vi "Project-SmartHome.vi"() -> ()   [LabVIEW 2013] (continued)
      }
      event Value Change {
        # "Air conditional - Bed room (set temperature)"
        n177 = event-data() -> ()  [unwired: 1 in, 6 out]
        n178 = Decimal String To Number(string="String") -> (number=w653:i32)  [unwired: 2 in, 1 out]
        n179 = Type Cast(x=6.0) -> (*(type *) &x=w659:string)  [unwired: 1 in]
        n180 = TCP Write(connection ID=w658, data in=w659, error in (no error)=w657) -> (connection ID out=w661:refnum<k5>, error out=w662:errorcluster)  [unwired: 1 in, 1 out]
        n181 = Bundle("?", w653, 1.0) -> (w663:cluster{bool, i32, dbl})  [unwired: 1 in]
        n182 = Type Cast(x=w663) -> (*(type *) &x=w665:string)  [unwired: 1 in]
        n183 = TCP Write(connection ID=w661, data in=w665, error in (no error)=w662) -> (connection ID out=w656:refnum<k5>, error out=w655:errorcluster)  [unwired: 1 in, 1 out]
      }
      event Value Change {
        n184 = event-data() -> ()  [unwired: 1 in, 6 out]
        n185 = Type Cast(x=0.0) -> (*(type *) &x=w671:string)  [unwired: 1 in]
        n186 = TCP Write(connection ID=w668, data in=w671, error in (no error)=w669) -> (connection ID out=w667:refnum<k5>, error out=w666:errorcluster)  [unwired: 1 in, 1 out]
        n187 = Bundle("?", 15.0) -> (w675:cluster{bool, dbl})  [unwired: 1 in]
        n188 = Type Cast(x=w675) -> (*(type *) &x=w677:string)  [unwired: 1 in]
        n189 = TCP Write(connection ID=w667, data in=w677, error in (no error)=w666) -> (connection ID out=w674:refnum<k5>, error out=w673:errorcluster)  [unwired: 1 in, 1 out]
      }
      event "OK Button 18": Value Change {
        n190 = event-data() -> ()  [unwired: 1 in, 6 out]
        n191 = Type Cast(x=0.0) -> (*(type *) &x=w683:string)  [unwired: 1 in]
        n192 = TCP Write(connection ID=w680, data in=w683, error in (no error)=w681) -> (connection ID out=w679:refnum<k5>, error out=w678:errorcluster)  [unwired: 1 in, 1 out]
        n193 = Bundle("OK Button 18"="OK Button 18", 16.0) -> (w687:cluster{"OK Button 18":bool, dbl})  [unwired: 1 in]
        n194 = Type Cast(x=w687) -> (*(type *) &x=w689:string)  [unwired: 1 in]
        n195 = TCP Write(connection ID=w679, data in=w689, error in (no error)=w678) -> (connection ID out=w686:refnum<k5>, error out=w685:errorcluster)  [unwired: 1 in, 1 out]
      }
      event Value Change {
        # "Air conditional - Bedroom 2"
        n196 = event-data() -> ()  [unwired: 1 in, 6 out]
        n197 = property on="Tab Control" class="TabCtl (strict)"("Visible"=FALSE) -> ()  [unwired: 2 in, 2 out]
        n198 = property on="Tab Control 2" class="TabCtl (strict)"("Visible"=FALSE) -> ()  [unwired: 2 in, 2 out]
        n199 = property on="Tab Control 3" class="TabCtl (strict)"("Visible"=FALSE) -> ()  [unwired: 2 in, 2 out]
        n200 = property on="Tab Control 4" class="TabCtl (strict)"("Visible"=FALSE) -> ()  [unwired: 2 in, 2 out]
        n201 = property on="Tab Control 5" class="TabCtl (strict)"("Visible"=FALSE) -> ()  [unwired: 2 in, 2 out]
        n202 = property on="Tab Control 11" class="TabCtl (strict)"("Visible"=FALSE) -> ()  [unwired: 2 in, 2 out]
        n203 = property on="Tab Control 6" class="TabCtl (strict)"("Visible"=FALSE) -> ()  [unwired: 2 in, 2 out]
        n204 = property on="Tab Control 10" class="TabCtl (strict)"("Visible"=FALSE) -> ()  [unwired: 2 in, 2 out]
        n205 = property on="Tab Control 13" class="TabCtl (strict)"("Visible"=FALSE) -> ()  [unwired: 2 in, 2 out]
        n206 = property on="Tab Control 7" class="TabCtl (strict)"("Visible"=FALSE) -> ()  [unwired: 2 in, 2 out]
        n207 = property on="Tab Control 12" class="TabCtl (strict)"("Visible"=FALSE) -> ()  [unwired: 2 in, 2 out]
        n208 = property on="Tab Control 8" class="TabCtl (strict)"("Visible"=FALSE) -> ()  [unwired: 2 in, 2 out]
        n209 = property on="Tab Control 9" class="TabCtl (strict)"("Visible"=FALSE) -> ()  [unwired: 2 in, 2 out]
        n210 = property on="Tab Control 24" class="TabCtl (strict)"("Visible"=FALSE) -> ()  [unwired: 2 in, 2 out]
        n211 = property on="Tab Control 15" class="TabCtl (strict)"("Visible"=FALSE) -> ()  [unwired: 2 in, 2 out]
        n212 = property on="Tab Control 21" class="TabCtl (strict)"("Visible"=TRUE) -> ()  [unwired: 2 in, 2 out]
        n213 = property on="Tab Control 16" class="TabCtl (strict)"("Visible"=FALSE) -> ()  [unwired: 2 in, 2 out]
        n214 = property on="Tab Control 17" class="TabCtl (strict)"("Visible"=FALSE) -> ()  [unwired: 2 in, 2 out]
        n215 = property on="Tab Control 22" class="TabCtl (strict)"("Visible"=FALSE) -> ()  [unwired: 2 in, 2 out]
        n216 = property on="Tab Control 23" class="TabCtl (strict)"("Visible"=FALSE) -> ()  [unwired: 2 in, 2 out]
        n217 = property on="Tab Control 18" class="TabCtl (strict)"("Visible"=FALSE) -> ()  [unwired: 2 in, 2 out]
        n218 = property on="Tab Control 19" class="TabCtl (strict)"("Visible"=FALSE) -> ()  [unwired: 2 in, 2 out]
        n219 = property on="Tab Control 14" class="TabCtl (strict)"("Visible"=FALSE) -> ()  [unwired: 2 in, 2 out]
      }
      event Value Change {
        n220 = event-data() -> ()  [unwired: 1 in, 6 out]
        n221 = Type Cast(x=0.0) -> (*(type *) &x=w718:string)  [unwired: 1 in]
        n222 = TCP Write(connection ID=w713, data in=w718, error in (no error)=w716) -> (connection ID out=w714:refnum<k5>, error out=w715:errorcluster)  [unwired: 1 in, 1 out]
        n223 = Bundle("?", 14.0) -> (w722:cluster{bool, dbl})  [unwired: 1 in]
        n224 = Type Cast(x=w722) -> (*(type *) &x=w724:string)  [unwired: 1 in]
        n225 = TCP Write(connection ID=w714, data in=w724, error in (no error)=w715) -> (connection ID out=w721:refnum<k5>, error out=w720:errorcluster)  [unwired: 1 in, 1 out]
      }
      event "OK Button 16": Value Change {
        n226 = event-data() -> ()  [unwired: 1 in, 6 out]
        n227 = Type Cast(x=0.0) -> (*(type *) &x=w730:string)  [unwired: 1 in]
        n228 = TCP Write(connection ID=w728, data in=w730, error in (no error)=w725) -> (connection ID out=w727:refnum<k5>, error out=w726:errorcluster)  [unwired: 1 in, 1 out]
        n229 = Bundle("OK Button 16"="OK Button 16", 20.0) -> (w734:cluster{"OK Button 16":bool, dbl})  [unwired: 1 in]
        n230 = Type Cast(x=w734) -> (*(type *) &x=w736:string)  [unwired: 1 in]
        n231 = TCP Write(connection ID=w727, data in=w736, error in (no error)=w726) -> (connection ID out=w733:refnum<k5>, error out=w732:errorcluster)  [unwired: 1 in, 1 out]
      }
      event Value Change {
        n232 = event-data() -> ()  [unwired: 1 in, 6 out]
        n233 = Type Cast(x=2.0) -> (*(type *) &x=w750:string)  [unwired: 1 in]
        n234 = TCP Write(connection ID=w741, data in=w750, error in (no error)=w740) -> (connection ID out=w748:refnum<k5>, error out=w747:errorcluster)  [unwired: 1 in, 1 out]
        n235 = Decimal String To Number(string="String") -> (number=w751:i32)  [unwired: 2 in, 1 out]
        n236 = Bundle(w751, 24.0, "?", 1.0) -> (w746:cluster{i32, dbl, bool, dbl})  [unwired: 1 in]
        n237 = Type Cast(x=w746) -> (*(type *) &x=w744:string)  [unwired: 1 in]
        n238 = TCP Write(connection ID=w748, data in=w744, error in (no error)=w747) -> (connection ID out=w742:refnum<k5>, error out=w743:errorcluster)  [unwired: 1 in, 1 out]
      }
      event Value Change {
        (unwired) FALSE ("Visible")
        n239 = event-data() -> ()  [unwired: 1 in, 6 out]
        n240 = property on="Tab Control 18" class="TabCtl (strict)"("Visible"=FALSE) -> ()  [unwired: 2 in, 2 out]
        n241 = property on="Tab Control 17" class="TabCtl (strict)"("Visible"=FALSE) -> ()  [unwired: 2 in, 2 out]
        n242 = property on="Tab Control 10" class="TabCtl (strict)"("Visible"=FALSE) -> ()  [unwired: 2 in, 2 out]
        n243 = property on="Tab Control 11" class="TabCtl (strict)"("Visible"=FALSE) -> ()  [unwired: 2 in, 2 out]
        n244 = property on="Tab Control 6" class="TabCtl (strict)"("Visible"=FALSE) -> ()  [unwired: 2 in, 2 out]
        n245 = property on="Tab Control 5" class="TabCtl (strict)"("Visible"=FALSE) -> ()  [unwired: 2 in, 2 out]
        n246 = property on="Tab Control 22" class="TabCtl (strict)"("Visible"=FALSE) -> ()  [unwired: 2 in, 2 out]
        n247 = property on="Tab Control 2" class="TabCtl (strict)"("Visible"=FALSE) -> ()  [unwired: 2 in, 2 out]
        n248 = property on="Tab Control 3" class="TabCtl (strict)"("Visible"=TRUE) -> ()  [unwired: 2 in, 2 out]
        n249 = property on="Tab Control 12" class="TabCtl (strict)"("Visible"=FALSE) -> ()  [unwired: 2 in, 2 out]
        n250 = property on="Tab Control 21" class="TabCtl (strict)"("Visible"=FALSE) -> ()  [unwired: 2 in, 2 out]
        n251 = property on="Tab Control 19" class="TabCtl (strict)"("Visible"=FALSE) -> ()  [unwired: 2 in, 2 out]
        n252 = property on="Tab Control 8" class="TabCtl (strict)"("Visible"=FALSE) -> ()  [unwired: 2 in, 2 out]
        n253 = property on="Tab Control 7" class="TabCtl (strict)"("Visible"=FALSE) -> ()  [unwired: 2 in, 2 out]
        n254 = property on="Tab Control 4" class="TabCtl (strict)"("Visible"=FALSE) -> ()  [unwired: 2 in, 2 out]
        n255 = property on="Tab Control 9" class="TabCtl (strict)"("Visible"=FALSE) -> ()  [unwired: 2 in, 2 out]
        n256 = property on="Tab Control" class="TabCtl (strict)"("Visible"=FALSE) -> ()  [unwired: 2 in, 2 out]
        n257 = property on="Tab Control 14" class="TabCtl (strict)"("Visible"=FALSE) -> ()  [unwired: 2 in, 2 out]
        n258 = property on="Tab Control 13" class="TabCtl (strict)"("Visible"=FALSE) -> ()  [unwired: 2 in, 2 out]
        n259 = property on="Tab Control 16" class="TabCtl (strict)"("Visible"=FALSE) -> ()  [unwired: 2 in, 2 out]
        n260 = property on="Tab Control 24" class="TabCtl (strict)"("Visible"=FALSE) -> ()  [unwired: 2 in, 2 out]
        n261 = property on="Tab Control 15" class="TabCtl (strict)"("Visible"=FALSE) -> ()  [unwired: 2 in, 2 out]
      }
      event Value Change {
        # "Air conditional - Bed room"
        n262 = event-data() -> ()  [unwired: 1 in, 6 out]
        n263 = local read item#4() -> (w774:dbl)
        n264 = Type Cast(x=5.0) -> (*(type *) &x=w780:string)  [unwired: 1 in]
        n265 = TCP Write(connection ID=w778, data in=w780, error in (no error)=w777) -> (connection ID out=w782:refnum<k5>, error out=w783:errorcluster)  [unwired: 1 in, 1 out]
        n266 = Bundle("?", w774, 3.0) -> (w784:cluster{bool, dbl, dbl})  [unwired: 1 in]
        n267 = Type Cast(x=w784) -> (*(type *) &x=w786:string)  [unwired: 1 in]
        n268 = TCP Write(connection ID=w782, data in=w786, error in (no error)=w783) -> (connection ID out=w776:refnum<k5>, error out=w775:errorcluster)  [unwired: 1 in, 1 out]
      }
      event Value Change {
        n269 = event-data() -> ()  [unwired: 1 in, 6 out]
        n270 = property on="Tab Control 18" class="TabCtl (strict)"("Visible"=FALSE) -> ()  [unwired: 2 in, 2 out]
        n271 = property on="Tab Control 17" class="TabCtl (strict)"("Visible"=FALSE) -> ()  [unwired: 2 in, 2 out]
        n272 = property on="Tab Control 10" class="TabCtl (strict)"("Visible"=FALSE) -> ()  [unwired: 2 in, 2 out]
        n273 = property on="Tab Control 6" class="TabCtl (strict)"("Visible"=FALSE) -> ()  [unwired: 2 in, 2 out]
        n274 = property on="Tab Control 5" class="TabCtl (strict)"("Visible"=FALSE) -> ()  [unwired: 2 in, 2 out]
        n275 = property on="Tab Control 2" class="TabCtl (strict)"("Visible"=FALSE) -> ()  [unwired: 2 in, 2 out]
        n276 = property on="Tab Control 3" class="TabCtl (strict)"("Visible"=FALSE) -> ()  [unwired: 2 in, 2 out]
        n277 = property on="Tab Control 22" class="TabCtl (strict)"("Visible"=FALSE) -> ()  [unwired: 2 in, 2 out]
        n278 = property on="Tab Control 12" class="TabCtl (strict)"("Visible"=FALSE) -> ()  [unwired: 2 in, 2 out]
        n279 = property on="Tab Control 8" class="TabCtl (strict)"("Visible"=FALSE) -> ()  [unwired: 2 in, 2 out]
        n280 = property on="Tab Control 7" class="TabCtl (strict)"("Visible"=FALSE) -> ()  [unwired: 2 in, 2 out]
        n281 = property on="Tab Control 4" class="TabCtl (strict)"("Visible"=FALSE) -> ()  [unwired: 2 in, 2 out]
        n282 = property on="Tab Control 21" class="TabCtl (strict)"("Visible"=FALSE) -> ()  [unwired: 2 in, 2 out]
        n283 = property on="Tab Control 9" class="TabCtl (strict)"("Visible"=FALSE) -> ()  [unwired: 2 in, 2 out]
        n284 = property on="Tab Control" class="TabCtl (strict)"("Visible"=FALSE) -> ()  [unwired: 2 in, 2 out]
        n285 = property on="Tab Control 11" class="TabCtl (strict)"("Visible"=FALSE) -> ()  [unwired: 2 in, 2 out]
        n286 = property on="Tab Control 19" class="TabCtl (strict)"("Visible"=FALSE) -> ()  [unwired: 2 in, 2 out]
        n287 = property on="Tab Control 24" class="TabCtl (strict)"("Visible"=FALSE) -> ()  [unwired: 2 in, 2 out]
        n288 = property on="Tab Control 16" class="TabCtl (strict)"("Visible"=TRUE) -> ()  [unwired: 2 in, 2 out]
        n289 = property on="Tab Control 14" class="TabCtl (strict)"("Visible"=FALSE) -> ()  [unwired: 2 in, 2 out]
        n290 = property on="Tab Control 13" class="TabCtl (strict)"("Visible"=FALSE) -> ()  [unwired: 2 in, 2 out]
        n291 = property on="Tab Control 15" class="TabCtl (strict)"("Visible"=FALSE) -> ()  [unwired: 2 in, 2 out]
      }
      event Value Change {
        n292 = event-data() -> ()  [unwired: 1 in, 6 out]
        n293 = property on="Tab Control 18" class="TabCtl (strict)"("Visible"=FALSE) -> ()  [unwired: 2 in, 2 out]
        n294 = property on="Tab Control 17" class="TabCtl (strict)"("Visible"=FALSE) -> ()  [unwired: 2 in, 2 out]
        n295 = property on="Tab Control 10" class="TabCtl (strict)"("Visible"=FALSE) -> ()  [unwired: 2 in, 2 out]
        n296 = property on="Tab Control 6" class="TabCtl (strict)"("Visible"=FALSE) -> ()  [unwired: 2 in, 2 out]
        n297 = property on="Tab Control 24" class="TabCtl (strict)"("Visible"=FALSE) -> ()  [unwired: 2 in, 2 out]
        n298 = property on="Tab Control 5" class="TabCtl (strict)"("Visible"=FALSE) -> ()  [unwired: 2 in, 2 out]
        n299 = property on="Tab Control 2" class="TabCtl (strict)"("Visible"=FALSE) -> ()  [unwired: 2 in, 2 out]
        n300 = property on="Tab Control 22" class="TabCtl (strict)"("Visible"=FALSE) -> ()  [unwired: 2 in, 2 out]
        n301 = property on="Tab Control 3" class="TabCtl (strict)"("Visible"=FALSE) -> ()  [unwired: 2 in, 2 out]
        n302 = property on="Tab Control 12" class="TabCtl (strict)"("Visible"=FALSE) -> ()  [unwired: 2 in, 2 out]
        n303 = property on="Tab Control 8" class="TabCtl (strict)"("Visible"=FALSE) -> ()  [unwired: 2 in, 2 out]
        n304 = property on="Tab Control 7" class="TabCtl (strict)"("Visible"=FALSE) -> ()  [unwired: 2 in, 2 out]
        n305 = property on="Tab Control 4" class="TabCtl (strict)"("Visible"=FALSE) -> ()  [unwired: 2 in, 2 out]
        n306 = property on="Tab Control 9" class="TabCtl (strict)"("Visible"=FALSE) -> ()  [unwired: 2 in, 2 out]
        n307 = property on="Tab Control 21" class="TabCtl (strict)"("Visible"=FALSE) -> ()  [unwired: 2 in, 2 out]
        n308 = property on="Tab Control" class="TabCtl (strict)"("Visible"=FALSE) -> ()  [unwired: 2 in, 2 out]
        n309 = property on="Tab Control 19" class="TabCtl (strict)"("Visible"=FALSE) -> ()  [unwired: 2 in, 2 out]
        n310 = property on="Tab Control 11" class="TabCtl (strict)"("Visible"=TRUE) -> ()  [unwired: 2 in, 2 out]
        n311 = property on="Tab Control 16" class="TabCtl (strict)"("Visible"=FALSE) -> ()  [unwired: 2 in, 2 out]
        n312 = property on="Tab Control 14" class="TabCtl (strict)"("Visible"=FALSE) -> ()  [unwired: 2 in, 2 out]
        n313 = property on="Tab Control 13" class="TabCtl (strict)"("Visible"=FALSE) -> ()  [unwired: 2 in, 2 out]
        n314 = property on="Tab Control 15" class="TabCtl (strict)"("Visible"=FALSE) -> ()  [unwired: 2 in, 2 out]
      }
      event "Back 10": Value Change {
        n315 = event-data() -> ()  [unwired: 1 in, 6 out]
        n316 = property on="Tab Control 11" class="TabCtl (strict)"("Visible"=FALSE) -> ()  [unwired: 2 in, 2 out]
        n317 = property on="Tab Control 16" class="TabCtl (strict)"("Visible"=TRUE) -> ()  [unwired: 2 in, 2 out]
      }
      event "Back 11": Value Change {
        n318 = event-data() -> ()  [unwired: 1 in, 6 out]
        n319 = property on="Tab Control 17" class="TabCtl (strict)"("Visible"=FALSE) -> ()  [unwired: 2 in, 2 out]
        n320 = property on="Tab Control 16" class="TabCtl (strict)"("Visible"=TRUE) -> ()  [unwired: 2 in, 2 out]
      }
      event "Back 12": Value Change {
        n321 = event-data() -> ()  [unwired: 1 in, 6 out]
        n322 = property on="Tab Control 18" class="TabCtl (strict)"("Visible"=FALSE) -> ()  [unwired: 2 in, 2 out]
        n323 = property on="Tab Control 16" class="TabCtl (strict)"("Visible"=TRUE) -> ()  [unwired: 2 in, 2 out]
      }
      event "Back 13": Value Change {
        n324 = event-data() -> ()  [unwired: 1 in, 6 out]
        n325 = property on="Tab Control 12" class="TabCtl (strict)"("Visible"=FALSE) -> ()  [unwired: 2 in, 2 out]
        n326 = property on="Tab Control 2" class="TabCtl (strict)"("Visible"=TRUE) -> ()  [unwired: 2 in, 2 out]
      }
      event Value Change {
        n327 = event-data() -> ()  [unwired: 1 in, 6 out]
        n328 = Type Cast(x=2.0) -> (*(type *) &x=w846:string)  [unwired: 1 in]
        n329 = TCP Write(connection ID=w842, data in=w846, error in (no error)=w841) -> (connection ID out=w848:refnum<k5>, error out=w849:errorcluster)  [unwired: 1 in, 1 out]
        n330 = Decimal String To Number(string="String") -> (number=w845:i32)  [unwired: 2 in, 1 out]
        n331 = Bundle(w845, 23.0, "?") -> (w850:cluster{i32, dbl, bool})  [unwired: 1 in]
        n332 = Type Cast(x=w850) -> (*(type *) &x=w852:string)  [unwired: 1 in]
        n333 = TCP Write(connection ID=w848, data in=w852, error in (no error)=w849) -> (connection ID out=w843:refnum<k5>, error out=w844:errorcluster)  [unwired: 1 in, 1 out]
      }
      event Value Change {
        n334 = event-data() -> ()  [unwired: 1 in, 6 out]
        n335 = property on="Tab Control 18" class="TabCtl (strict)"("Visible"=FALSE) -> ()  [unwired: 2 in, 2 out]
        n336 = property on="Tab Control 17" class="TabCtl (strict)"("Visible"=TRUE) -> ()  [unwired: 2 in, 2 out]
        n337 = property on="Tab Control 10" class="TabCtl (strict)"("Visible"=FALSE) -> ()  [unwired: 2 in, 2 out]
        n338 = property on="Tab Control 6" class="TabCtl (strict)"("Visible"=FALSE) -> ()  [unwired: 2 in, 2 out]
        n339 = property on="Tab Control 5" class="TabCtl (strict)"("Visible"=FALSE) -> ()  [unwired: 2 in, 2 out]
        n340 = property on="Tab Control 22" class="TabCtl (strict)"("Visible"=FALSE) -> ()  [unwired: 2 in, 2 out]
        n341 = property on="Tab Control 2" class="TabCtl (strict)"("Visible"=FALSE) -> ()  [unwired: 2 in, 2 out]
        n342 = property on="Tab Control 3" class="TabCtl (strict)"("Visible"=FALSE) -> ()  [unwired: 2 in, 2 out]
        n343 = property on="Tab Control 21" class="TabCtl (strict)"("Visible"=FALSE) -> ()  [unwired: 2 in, 2 out]
        n344 = property on="Tab Control 12" class="TabCtl (strict)"("Visible"=FALSE) -> ()  [unwired: 2 in, 2 out]
        n345 = property on="Tab Control 8" class="TabCtl (strict)"("Visible"=FALSE) -> ()  [unwired: 2 in, 2 out]
        n346 = property on="Tab Control 7" class="TabCtl (strict)"("Visible"=FALSE) -> ()  [unwired: 2 in, 2 out]
        n347 = property on="Tab Control 4" class="TabCtl (strict)"("Visible"=FALSE) -> ()  [unwired: 2 in, 2 out]
        n348 = property on="Tab Control 9" class="TabCtl (strict)"("Visible"=FALSE) -> ()  [unwired: 2 in, 2 out]
        n349 = property on="Tab Control" class="TabCtl (strict)"("Visible"=FALSE) -> ()  [unwired: 2 in, 2 out]
        n350 = property on="Tab Control 11" class="TabCtl (strict)"("Visible"=FALSE) -> ()  [unwired: 2 in, 2 out]
        n351 = property on="Tab Control 19" class="TabCtl (strict)"("Visible"=FALSE) -> ()  [unwired: 2 in, 2 out]
        n352 = property on="Tab Control 24" class="TabCtl (strict)"("Visible"=FALSE) -> ()  [unwired: 2 in, 2 out]
        n353 = property on="Tab Control 16" class="TabCtl (strict)"("Visible"=FALSE) -> ()  [unwired: 2 in, 2 out]
        n354 = property on="Tab Control 14" class="TabCtl (strict)"("Visible"=FALSE) -> ()  [unwired: 2 in, 2 out]
        n355 = property on="Tab Control 13" class="TabCtl (strict)"("Visible"=FALSE) -> ()  [unwired: 2 in, 2 out]
        n356 = property on="Tab Control 15" class="TabCtl (strict)"("Visible"=FALSE) -> ()  [unwired: 2 in, 2 out]
      }
      event Value Change {
        n357 = event-data() -> ()  [unwired: 1 in, 6 out]
        n358 = property on="Tab Control 18" class="TabCtl (strict)"("Visible"=TRUE) -> ()  [unwired: 2 in, 2 out]
        n359 = property on="Tab Control 17" class="TabCtl (strict)"("Visible"=FALSE) -> ()  [unwired: 2 in, 2 out]
        n360 = property on="Tab Control 24" class="TabCtl (strict)"("Visible"=FALSE) -> ()  [unwired: 2 in, 2 out]
        n361 = property on="Tab Control 10" class="TabCtl (strict)"("Visible"=FALSE) -> ()  [unwired: 2 in, 2 out]
        n362 = property on="Tab Control 6" class="TabCtl (strict)"("Visible"=FALSE) -> ()  [unwired: 2 in, 2 out]
        n363 = property on="Tab Control 5" class="TabCtl (strict)"("Visible"=FALSE) -> ()  [unwired: 2 in, 2 out]
        n364 = property on="Tab Control 22" class="TabCtl (strict)"("Visible"=FALSE) -> ()  [unwired: 2 in, 2 out]
        n365 = property on="Tab Control 2" class="TabCtl (strict)"("Visible"=FALSE) -> ()  [unwired: 2 in, 2 out]
        n366 = property on="Tab Control 3" class="TabCtl (strict)"("Visible"=FALSE) -> ()  [unwired: 2 in, 2 out]
        n367 = property on="Tab Control 12" class="TabCtl (strict)"("Visible"=FALSE) -> ()  [unwired: 2 in, 2 out]
        n368 = property on="Tab Control 8" class="TabCtl (strict)"("Visible"=FALSE) -> ()  [unwired: 2 in, 2 out]
        n369 = property on="Tab Control 7" class="TabCtl (strict)"("Visible"=FALSE) -> ()  [unwired: 2 in, 2 out]
        n370 = property on="Tab Control 4" class="TabCtl (strict)"("Visible"=FALSE) -> ()  [unwired: 2 in, 2 out]
        n371 = property on="Tab Control 9" class="TabCtl (strict)"("Visible"=FALSE) -> ()  [unwired: 2 in, 2 out]
        n372 = property on="Tab Control" class="TabCtl (strict)"("Visible"=FALSE) -> ()  [unwired: 2 in, 2 out]
        n373 = property on="Tab Control 21" class="TabCtl (strict)"("Visible"=FALSE) -> ()  [unwired: 2 in, 2 out]
        n374 = property on="Tab Control 11" class="TabCtl (strict)"("Visible"=FALSE) -> ()  [unwired: 2 in, 2 out]
        n375 = property on="Tab Control 19" class="TabCtl (strict)"("Visible"=FALSE) -> ()  [unwired: 2 in, 2 out]
        n376 = property on="Tab Control 16" class="TabCtl (strict)"("Visible"=FALSE) -> ()  [unwired: 2 in, 2 out]
        n377 = property on="Tab Control 14" class="TabCtl (strict)"("Visible"=FALSE) -> ()  [unwired: 2 in, 2 out]
        n378 = property on="Tab Control 13" class="TabCtl (strict)"("Visible"=FALSE) -> ()  [unwired: 2 in, 2 out]
        n379 = property on="Tab Control 15" class="TabCtl (strict)"("Visible"=FALSE) -> ()  [unwired: 2 in, 2 out]
      }
      event Value Change {
        n380 = event-data() -> ()  [unwired: 1 in, 6 out]
        n381 = Type Cast(x=1.0) -> (*(type *) &x=w897:string)  [unwired: 1 in]
        n382 = TCP Write(connection ID=w900, data in=w897, error in (no error)=w899) -> (connection ID out=w901:refnum<k5>, error out=w902:errorcluster)  [unwired: 1 in, 1 out]
        n383 = Bundle("?", 19.0) -> (w906:cluster{dbl, dbl})  [unwired: 1 in]
        n384 = Type Cast(x=w906) -> (*(type *) &x=w908:string)  [unwired: 1 in]
        n385 = TCP Write(connection ID=w901, data in=w908, error in (no error)=w902) -> (connection ID out=w904:refnum<k5>, error out=w903:errorcluster)  [unwired: 1 in, 1 out]
      }
      event Value Change {
        n386 = event-data() -> ()  [unwired: 1 in, 6 out]
        n387 = Type Cast(x=1.0) -> (*(type *) &x=w914:string)  [unwired: 1 in]
        n388 = TCP Write(connection ID=w911, data in=w914, error in (no error)=w910) -> (connection ID out=w916:refnum<k5>, error out=w917:errorcluster)  [unwired: 1 in, 1 out]
        n389 = Bundle("?", 21.0) -> (w918:cluster{dbl, dbl})  [unwired: 1 in]
        n390 = Type Cast(x=w918) -> (*(type *) &x=w920:string)  [unwired: 1 in]
        n391 = TCP Write(connection ID=w916, data in=w920, error in (no error)=w917) -> (connection ID out=w912:refnum<k5>, error out=w913:errorcluster)  [unwired: 1 in, 1 out]
      }
      event Value Change {
        n392 = event-data() -> ()  [unwired: 1 in, 6 out]
        n393 = Type Cast(x=1.0) -> (*(type *) &x=w926:string)  [unwired: 1 in]
        n394 = TCP Write(connection ID=w923, data in=w926, error in (no error)=w924) -> (connection ID out=w928:refnum<k5>, error out=w929:errorcluster)  [unwired: 1 in, 1 out]
        n395 = Bundle("?", 20.0) -> (w930:cluster{dbl, dbl})  [unwired: 1 in]
        n396 = Type Cast(x=w930) -> (*(type *) &x=w932:string)  [unwired: 1 in]
        n397 = TCP Write(connection ID=w928, data in=w932, error in (no error)=w929) -> (connection ID out=w922:refnum<k5>, error out=w921:errorcluster)  [unwired: 1 in, 1 out]
      }
      event Value Change {
        n398 = event-data() -> ()  [unwired: 1 in, 6 out]
        n399 = Type Cast(x=2.0) -> (*(type *) &x=w940:string)  [unwired: 1 in]
        n400 = TCP Write(connection ID=w937, data in=w940, error in (no error)=w936) -> (connection ID out=w942:refnum<k5>, error out=w943:errorcluster)  [unwired: 1 in, 1 out]
        n401 = Decimal String To Number(string="String") -> (number=w934:i32)  [unwired: 2 in, 1 out]
        n402 = Bundle(w934, 22.0, "?") -> (w944:cluster{i32, dbl, bool})  [unwired: 1 in]
        n403 = Type Cast(x=w944) -> (*(type *) &x=w946:string)  [unwired: 1 in]
        n404 = TCP Write(connection ID=w942, data in=w946, error in (no error)=w943) -> (connection ID out=w939:refnum<k5>, error out=w938:errorcluster)  [unwired: 1 in, 1 out]
      }
      event Value Change {
        (unwired) FALSE ("Visible")
        n405 = event-data() -> ()  [unwired: 1 in, 6 out]
        n406 = property on="Tab Control 18" class="TabCtl (strict)"("Visible"=FALSE) -> ()  [unwired: 2 in, 2 out]
        n407 = property on="Tab Control 17" class="TabCtl (strict)"("Visible"=FALSE) -> ()  [unwired: 2 in, 2 out]
        n408 = property on="Tab Control 6" class="TabCtl (strict)"("Visible"=FALSE) -> ()  [unwired: 2 in, 2 out]
        n409 = property on="Tab Control 10" class="TabCtl (strict)"("Visible"=FALSE) -> ()  [unwired: 2 in, 2 out]
        n410 = property on="Tab Control 8" class="TabCtl (strict)"("Visible"=FALSE) -> ()  [unwired: 2 in, 2 out]
        n411 = property on="Tab Control 9" class="TabCtl (strict)"("Visible"=FALSE) -> ()  [unwired: 2 in, 2 out]
        n412 = property on="Tab Control 19" class="TabCtl (strict)"("Visible"=FALSE) -> ()  [unwired: 2 in, 2 out]
        n413 = property on="Tab Control 5" class="TabCtl (strict)"("Visible"=FALSE) -> ()  [unwired: 2 in, 2 out]
        n414 = property on="Tab Control 22" class="TabCtl (strict)"("Visible"=FALSE) -> ()  [unwired: 2 in, 2 out]
        n415 = property on="Tab Control 7" class="TabCtl (strict)"("Visible"=FALSE) -> ()  [unwired: 2 in, 2 out]
        n416 = property on="Tab Control 12" class="TabCtl (strict)"("Visible"=FALSE) -> ()  [unwired: 2 in, 2 out]
        n417 = property on="Tab Control 21" class="TabCtl (strict)"("Visible"=FALSE) -> ()  [unwired: 2 in, 2 out]
        n418 = property on="Tab Control 11" class="TabCtl (strict)"("Visible"=FALSE) -> ()  [unwired: 2 in, 2 out]
        n419 = property on="Tab Control 4" class="TabCtl (strict)"("Visible"=TRUE) -> ()  [unwired: 2 in, 2 out]
        n420 = property on="Tab Control 3" class="TabCtl (strict)"("Visible"=FALSE) -> ()  [unwired: 2 in, 2 out]
        n421 = property on="Tab Control" class="TabCtl (strict)"("Visible"=FALSE) -> ()  [unwired: 2 in, 2 out]
        n422 = property on="Tab Control 2" class="TabCtl (strict)"("Visible"=FALSE) -> ()  [unwired: 2 in, 2 out]
        n423 = property on="Tab Control 14" class="TabCtl (strict)"("Visible"=FALSE) -> ()  [unwired: 2 in, 2 out]
        n424 = property on="Tab Control 13" class="TabCtl (strict)"("Visible"=FALSE) -> ()  [unwired: 2 in, 2 out]
        n425 = property on="Tab Control 24" class="TabCtl (strict)"("Visible"=FALSE) -> ()  [unwired: 2 in, 2 out]
        n426 = property on="Tab Control 15" class="TabCtl (strict)"("Visible"=FALSE) -> ()  [unwired: 2 in, 2 out]
        n427 = property on="Tab Control 16" class="TabCtl (strict)"("Visible"=FALSE) -> ()  [unwired: 2 in, 2 out]
      }
      event "Back 3": Value Change {
        n428 = event-data() -> ()  [unwired: 1 in, 6 out]
        n429 = property on="Tab Control 4" class="TabCtl (strict)"("Visible"=FALSE) -> ()  [unwired: 2 in, 2 out]
        n430 = property on="Tab Control 3" class="TabCtl (strict)"("Visible"=TRUE) -> ()  [unwired: 2 in, 2 out]
      }
      event "Back 4": Value Change {
        n431 = event-data() -> ()  [unwired: 1 in, 6 out]
        n432 = property on="Tab Control 5" class="TabCtl (strict)"("Visible"=FALSE) -> ()  [unwired: 2 in, 2 out]
        n433 = property on="Tab Control 3" class="TabCtl (strict)"("Visible"=TRUE) -> ()  [unwired: 2 in, 2 out]
      }
      event "Back 5": Value Change {
        n434 = event-data() -> ()  [unwired: 1 in, 6 out]
        n435 = property on="Tab Control 6" class="TabCtl (strict)"("Visible"=FALSE) -> ()  [unwired: 2 in, 2 out]
        n436 = property on="Tab Control 3" class="TabCtl (strict)"("Visible"=TRUE) -> ()  [unwired: 2 in, 2 out]
      }
      event "Back 6": Value Change {
        n437 = event-data() -> ()  [unwired: 1 in, 6 out]
        n438 = property on="Tab Control 7" class="TabCtl (strict)"("Visible"=FALSE) -> ()  [unwired: 2 in, 2 out]
        n439 = property on="Tab Control 3" class="TabCtl (strict)"("Visible"=TRUE) -> ()  [unwired: 2 in, 2 out]
      }
      event "Back 7": Value Change {
        n440 = event-data() -> ()  [unwired: 1 in, 6 out]
        n441 = property on="Tab Control 8" class="TabCtl (strict)"("Visible"=FALSE) -> ()  [unwired: 2 in, 2 out]
        n442 = property on="Tab Control 3" class="TabCtl (strict)"("Visible"=TRUE) -> ()  [unwired: 2 in, 2 out]
      }
      event "Back 8": Value Change {
        n443 = event-data() -> ()  [unwired: 1 in, 6 out]
        n444 = property on="Tab Control 9" class="TabCtl (strict)"("Visible"=FALSE) -> ()  [unwired: 2 in, 2 out]
        n445 = property on="Tab Control 3" class="TabCtl (strict)"("Visible"=TRUE) -> ()  [unwired: 2 in, 2 out]
      }
      event "Back 9": Value Change {
        n446 = event-data() -> ()  [unwired: 1 in, 6 out]
        n447 = property on="Tab Control 16" class="TabCtl (strict)"("Visible"=FALSE) -> ()  [unwired: 2 in, 2 out]
        n448 = property on="Tab Control 2" class="TabCtl (strict)"("Visible"=TRUE) -> ()  [unwired: 2 in, 2 out]
      }
      event Value Change {
        n449 = event-data() -> ()  [unwired: 1 in, 6 out]
        n450 = property on="Tab Control 18" class="TabCtl (strict)"("Visible"=FALSE) -> ()  [unwired: 2 in, 2 out]
        n451 = property on="Tab Control 17" class="TabCtl (strict)"("Visible"=FALSE) -> ()  [unwired: 2 in, 2 out]
        n452 = property on="Tab Control 19" class="TabCtl (strict)"("Visible"=FALSE) -> ()  [unwired: 2 in, 2 out]
        n453 = property on="Tab Control 6" class="TabCtl (strict)"("Visible"=FALSE) -> ()  [unwired: 2 in, 2 out]
        n454 = property on="Tab Control 10" class="TabCtl (strict)"("Visible"=FALSE) -> ()  [unwired: 2 in, 2 out]
        n455 = property on="Tab Control 8" class="TabCtl (strict)"("Visible"=FALSE) -> ()  [unwired: 2 in, 2 out]
        n456 = property on="Tab Control 9" class="TabCtl (strict)"("Visible"=FALSE) -> ()  [unwired: 2 in, 2 out]
        n457 = property on="Tab Control 5" class="TabCtl (strict)"("Visible"=FALSE) -> ()  [unwired: 2 in, 2 out]
        n458 = property on="Tab Control 24" class="TabCtl (strict)"("Visible"=FALSE) -> ()  [unwired: 2 in, 2 out]
        n459 = property on="Tab Control 12" class="TabCtl (strict)"("Visible"=TRUE) -> ()  [unwired: 2 in, 2 out]
        n460 = property on="Tab Control 7" class="TabCtl (strict)"("Visible"=FALSE) -> ()  [unwired: 2 in, 2 out]
        n461 = property on="Tab Control 11" class="TabCtl (strict)"("Visible"=FALSE) -> ()  [unwired: 2 in, 2 out]
        n462 = property on="Tab Control 4" class="TabCtl (strict)"("Visible"=FALSE) -> ()  [unwired: 2 in, 2 out]
        n463 = property on="Tab Control 3" class="TabCtl (strict)"("Visible"=FALSE) -> ()  [unwired: 2 in, 2 out]
        n464 = property on="Tab Control" class="TabCtl (strict)"("Visible"=FALSE) -> ()  [unwired: 2 in, 2 out]
        n465 = property on="Tab Control 2" class="TabCtl (strict)"("Visible"=FALSE) -> ()  [unwired: 2 in, 2 out]
        n466 = property on="Tab Control 22" class="TabCtl (strict)"("Visible"=FALSE) -> ()  [unwired: 2 in, 2 out]
        n467 = property on="Tab Control 16" class="TabCtl (strict)"("Visible"=FALSE) -> ()  [unwired: 2 in, 2 out]
        n468 = property on="Tab Control 14" class="TabCtl (strict)"("Visible"=FALSE) -> ()  [unwired: 2 in, 2 out]
        n469 = property on="Tab Control 13" class="TabCtl (strict)"("Visible"=FALSE) -> ()  [unwired: 2 in, 2 out]
        n470 = property on="Tab Control 15" class="TabCtl (strict)"("Visible"=FALSE) -> ()  [unwired: 2 in, 2 out]
        n471 = property on="Tab Control 21" class="TabCtl (strict)"("Visible"=FALSE) -> ()  [unwired: 2 in, 2 out]
      }
      event Value Change {
        n472 = event-data() -> ()  [unwired: 1 in, 6 out]
        n473 = property on="Tab Control 14" class="TabCtl (strict)"("Visible"=FALSE) -> ()  [unwired: 2 in, 2 out]
        n474 = property on="Tab Control 13" class="TabCtl (strict)"("Visible"=TRUE) -> ()  [unwired: 2 in, 2 out]
        n475 = property on="Tab Control 19" class="TabCtl (strict)"("Visible"=FALSE) -> ()  [unwired: 2 in, 2 out]
        n476 = property on="Tab Control 6" class="TabCtl (strict)"("Visible"=FALSE) -> ()  [unwired: 2 in, 2 out]
        n477 = property on="Tab Control 15" class="TabCtl (strict)"("Visible"=FALSE) -> ()  [unwired: 2 in, 2 out]
        n478 = property on="Tab Control 10" class="TabCtl (strict)"("Visible"=FALSE) -> ()  [unwired: 2 in, 2 out]
        n479 = property on="Tab Control 8" class="TabCtl (strict)"("Visible"=FALSE) -> ()  [unwired: 2 in, 2 out]
        n480 = property on="Tab Control 9" class="TabCtl (strict)"("Visible"=FALSE) -> ()  [unwired: 2 in, 2 out]
        n481 = property on="Tab Control 5" class="TabCtl (strict)"("Visible"=FALSE) -> ()  [unwired: 2 in, 2 out]
        n482 = property on="Tab Control 22" class="TabCtl (strict)"("Visible"=FALSE) -> ()  [unwired: 2 in, 2 out]
        n483 = property on="Tab Control 12" class="TabCtl (strict)"("Visible"=FALSE) -> ()  [unwired: 2 in, 2 out]
        n484 = property on="Tab Control 7" class="TabCtl (strict)"("Visible"=FALSE) -> ()  [unwired: 2 in, 2 out]
        n485 = property on="Tab Control 11" class="TabCtl (strict)"("Visible"=FALSE) -> ()  [unwired: 2 in, 2 out]
        n486 = property on="Tab Control 4" class="TabCtl (strict)"("Visible"=FALSE) -> ()  [unwired: 2 in, 2 out]
        n487 = property on="Tab Control 3" class="TabCtl (strict)"("Visible"=FALSE) -> ()  [unwired: 2 in, 2 out]
        n488 = property on="Tab Control" class="TabCtl (strict)"("Visible"=FALSE) -> ()  [unwired: 2 in, 2 out]
        n489 = property on="Tab Control 2" class="TabCtl (strict)"("Visible"=FALSE) -> ()  [unwired: 2 in, 2 out]
        n490 = property on="Tab Control 24" class="TabCtl (strict)"("Visible"=FALSE) -> ()  [unwired: 2 in, 2 out]
        n491 = property on="Tab Control 16" class="TabCtl (strict)"("Visible"=FALSE) -> ()  [unwired: 2 in, 2 out]
        n492 = property on="Tab Control 21" class="TabCtl (strict)"("Visible"=FALSE) -> ()  [unwired: 2 in, 2 out]
        n493 = property on="Tab Control 18" class="TabCtl (strict)"("Visible"=FALSE) -> ()  [unwired: 2 in, 2 out]
        n494 = property on="Tab Control 17" class="TabCtl (strict)"("Visible"=FALSE) -> ()  [unwired: 2 in, 2 out]
      }
      event "Back 14": Value Change {
        n495 = event-data() -> ()  [unwired: 1 in, 6 out]
        n496 = property on="Tab Control 13" class="TabCtl (strict)"("Visible"=FALSE) -> ()  [unwired: 2 in, 2 out]
        n497 = property on="Tab Control 12" class="TabCtl (strict)"("Visible"=TRUE) -> ()  [unwired: 2 in, 2 out]
      }
      event "Back 15": Value Change {
        n498 = event-data() -> ()  [unwired: 1 in, 6 out]
        n499 = property on="Tab Control 14" class="TabCtl (strict)"("Visible"=FALSE) -> ()  [unwired: 2 in, 2 out]
        n500 = property on="Tab Control 12" class="TabCtl (strict)"("Visible"=TRUE) -> ()  [unwired: 2 in, 2 out]
      }
      event "Back 16": Value Change {
        n501 = event-data() -> ()  [unwired: 1 in, 6 out]
        n502 = property on="Tab Control 15" class="TabCtl (strict)"("Visible"=FALSE) -> ()  [unwired: 2 in, 2 out]
        n503 = property on="Tab Control 12" class="TabCtl (strict)"("Visible"=TRUE) -> ()  [unwired: 2 in, 2 out]
      }
      event "Back 17": Value Change {
        n504 = event-data() -> ()  [unwired: 1 in, 6 out]
        n505 = property on="Tab Control 19" class="TabCtl (strict)"("Visible"=FALSE) -> ()  [unwired: 2 in, 2 out]
        n506 = property on="Tab Control 2" class="TabCtl (strict)"("Visible"=TRUE) -> ()  [unwired: 2 in, 2 out]
      }
      event "Back 18": Value Change {
        n507 = event-data() -> ()  [unwired: 1 in, 6 out]
        n508 = property on="Tab Control 22" class="TabCtl (strict)"("Visible"=FALSE) -> ()  [unwired: 2 in, 2 out]
        n509 = property on="Tab Control 19" class="TabCtl (strict)"("Visible"=TRUE) -> ()  [unwired: 2 in, 2 out]
      }
      event "Back 19": Value Change {
        n510 = event-data() -> ()  [unwired: 1 in, 6 out]
        n511 = property on="Tab Control 23" class="TabCtl (strict)"("Visible"=FALSE) -> ()  [unwired: 2 in, 2 out]
        n512 = property on="Tab Control 19" class="TabCtl (strict)"("Visible"=TRUE) -> ()  [unwired: 2 in, 2 out]
      }
      event "Back 20": Value Change {
        n513 = event-data() -> ()  [unwired: 1 in, 6 out]
        n514 = property on="Tab Control 21" class="TabCtl (strict)"("Visible"=FALSE) -> ()  [unwired: 2 in, 2 out]
        n515 = property on="Tab Control 19" class="TabCtl (strict)"("Visible"=TRUE) -> ()  [unwired: 2 in, 2 out]
      }
      event "Back 21": Value Change {
        n516 = event-data() -> ()  [unwired: 1 in, 6 out]
        n517 = property on="Tab Control 24" class="TabCtl (strict)"("Visible"=FALSE) -> ()  [unwired: 2 in, 2 out]
        n518 = property on="Tab Control 2" class="TabCtl (strict)"("Visible"=TRUE) -> ()  [unwired: 2 in, 2 out]
      }
      event "Back 22": Value Change {
        n519 = event-data() -> ()  [unwired: 1 in, 6 out]
        n520 = property on="Tab Control 25" class="TabCtl (strict)"("Visible"=FALSE) -> ()  [unwired: 2 in, 2 out]
        n521 = property on="Tab Control 2" class="TabCtl (strict)"("Visible"=TRUE) -> ()  [unwired: 2 in, 2 out]
      }
      event Value Change {
        n522 = event-data() -> ()  [unwired: 1 in, 6 out]
        n523 = property on="Tab Control 6" class="TabCtl (strict)"("Visible"=FALSE) -> ()  [unwired: 2 in, 2 out]
        n524 = property on="Tab Control 19" class="TabCtl (strict)"("Visible"=FALSE) -> ()  [unwired: 2 in, 2 out]
        n525 = property on="Tab Control 10" class="TabCtl (strict)"("Visible"=FALSE) -> ()  [unwired: 2 in, 2 out]
        n526 = property on="Tab Control 8" class="TabCtl (strict)"("Visible"=FALSE) -> ()  [unwired: 2 in, 2 out]
        n527 = property on="Tab Control 9" class="TabCtl (strict)"("Visible"=FALSE) -> ()  [unwired: 2 in, 2 out]
        n528 = property on="Tab Control 5" class="TabCtl (strict)"("Visible"=FALSE) -> ()  [unwired: 2 in, 2 out]
        n529 = property on="Tab Control 24" class="TabCtl (strict)"("Visible"=FALSE) -> ()  [unwired: 2 in, 2 out]
        n530 = property on="Tab Control 12" class="TabCtl (strict)"("Visible"=FALSE) -> ()  [unwired: 2 in, 2 out]
        n531 = property on="Tab Control 7" class="TabCtl (strict)"("Visible"=FALSE) -> ()  [unwired: 2 in, 2 out]
        n532 = property on="Tab Control 11" class="TabCtl (strict)"("Visible"=FALSE) -> ()  [unwired: 2 in, 2 out]
        n533 = property on="Tab Control 4" class="TabCtl (strict)"("Visible"=FALSE) -> ()  [unwired: 2 in, 2 out]
        n534 = property on="Tab Control 3" class="TabCtl (strict)"("Visible"=FALSE) -> ()  [unwired: 2 in, 2 out]
        n535 = property on="Tab Control" class="TabCtl (strict)"("Visible"=FALSE) -> ()  [unwired: 2 in, 2 out]
        n536 = property on="Tab Control 21" class="TabCtl (strict)"("Visible"=FALSE) -> ()  [unwired: 2 in, 2 out]
        n537 = property on="Tab Control 2" class="TabCtl (strict)"("Visible"=FALSE) -> ()  [unwired: 2 in, 2 out]
        n538 = property on="Tab Control 22" class="TabCtl (strict)"("Visible"=FALSE) -> ()  [unwired: 2 in, 2 out]
        n539 = property on="Tab Control 14" class="TabCtl (strict)"("Visible"=TRUE) -> ()  [unwired: 2 in, 2 out]
        n540 = property on="Tab Control 13" class="TabCtl (strict)"("Visible"=FALSE) -> ()  [unwired: 2 in, 2 out]
        n541 = property on="Tab Control 15" class="TabCtl (strict)"("Visible"=FALSE) -> ()  [unwired: 2 in, 2 out]
        n542 = property on="Tab Control 18" class="TabCtl (strict)"("Visible"=FALSE) -> ()  [unwired: 2 in, 2 out]
        n543 = property on="Tab Control 17" class="TabCtl (strict)"("Visible"=FALSE) -> ()  [unwired: 2 in, 2 out]
      }
      event Value Change {
        # "Air conditional - Master room"
        n544 = event-data() -> ()  [unwired: 1 in, 6 out]
        n545 = local read item#8() -> (w1066:dbl)
        n546 = Type Cast(x=5.0) -> (*(type *) &x=w1072:string)  [unwired: 1 in]
        n547 = TCP Write(connection ID=w1068, data in=w1072, error in (no error)=w1067) -> (connection ID out=w1074:refnum<k5>, error out=w1075:errorcluster)  [unwired: 1 in, 1 out]
        n548 = Bundle("?", w1066, 2.0) -> (w1076:cluster{bool, dbl, dbl})  [unwired: 1 in]
        n549 = Type Cast(x=w1076) -> (*(type *) &x=w1078:string)  [unwired: 1 in]
        n550 = TCP Write(connection ID=w1074, data in=w1078, error in (no error)=w1075) -> (connection ID out=w1070:refnum<k5>, error out=w1069:errorcluster)  [unwired: 1 in, 1 out]
      }
      event Value Change {
        # "Air conditional - Master room (slider)"
        n551 = event-data() -> ()  [unwired: 1 in, 6 out]
        n552 = local read item#5() -> (w1083:bool)
        n553 = Type Cast(x=5.0) -> (*(type *) &x=w1085:string)  [unwired: 1 in]
        n554 = TCP Write(connection ID=w1079, data in=w1085, error in (no error)=w1080) -> (connection ID out=w1087:refnum<k5>, error out=w1088:errorcluster)  [unwired: 1 in, 1 out]
        n555 = Bundle(w1083, "?", 2.0) -> (w1089:cluster{bool, dbl, dbl})  [unwired: 1 in]
        n556 = Type Cast(x=w1089) -> (*(type *) &x=w1091:string)  [unwired: 1 in]
        n557 = TCP Write(connection ID=w1087, data in=w1091, error in (no error)=w1088) -> (connection ID out=w1082:refnum<k5>, error out=w1081:errorcluster)  [unwired: 1 in, 1 out]
      }
      event Value Change {
        # "Air conditional - Bed room  (slider)_"
        n558 = event-data() -> ()  [unwired: 1 in, 6 out]
        n559 = local read item#1() -> (w1094:bool)
        n560 = Type Cast(x=5.0) -> (*(type *) &x=w1098:string)  [unwired: 1 in]
        n561 = TCP Write(connection ID=w1096, data in=w1098, error in (no error)=w1095) -> (connection ID out=w1100:refnum<k5>, error out=w1101:errorcluster)  [unwired: 1 in, 1 out]
        n562 = Bundle(w1094, "?", 3.0) -> (w1102:cluster{bool, dbl, dbl})  [unwired: 1 in]
        n563 = Type Cast(x=w1102) -> (*(type *) &x=w1104:string)  [unwired: 1 in]
        n564 = TCP Write(connection ID=w1100, data in=w1104, error in (no error)=w1101) -> (connection ID out=w1093:refnum<k5>, error out=w1092:errorcluster)  [unwired: 1 in, 1 out]
      }
      event Value Change {
        n565 = event-data() -> ()  [unwired: 1 in, 6 out]
        n566 = property on="Tab Control" class="TabCtl (strict)"("Visible"=FALSE) -> ()  [unwired: 2 in, 2 out]
        n567 = property on="Tab Control 2" class="TabCtl (strict)"("Visible"=FALSE) -> ()  [unwired: 2 in, 2 out]
        n568 = property on="Tab Control 3" class="TabCtl (strict)"("Visible"=FALSE) -> ()  [unwired: 2 in, 2 out]
        n569 = property on="Tab Control 4" class="TabCtl (strict)"("Visible"=FALSE) -> ()  [unwired: 2 in, 2 out]
        n570 = property on="Tab Control 5" class="TabCtl (strict)"("Visible"=FALSE) -> ()  [unwired: 2 in, 2 out]
        n571 = property on="Tab Control 11" class="TabCtl (strict)"("Visible"=FALSE) -> ()  [unwired: 2 in, 2 out]
        n572 = property on="Tab Control 6" class="TabCtl (strict)"("Visible"=FALSE) -> ()  [unwired: 2 in, 2 out]
        n573 = property on="Tab Control 10" class="TabCtl (strict)"("Visible"=FALSE) -> ()  [unwired: 2 in, 2 out]
        n574 = property on="Tab Control 13" class="TabCtl (strict)"("Visible"=FALSE) -> ()  [unwired: 2 in, 2 out]
        n575 = property on="Tab Control 7" class="TabCtl (strict)"("Visible"=FALSE) -> ()  [unwired: 2 in, 2 out]
        n576 = property on="Tab Control 12" class="TabCtl (strict)"("Visible"=FALSE) -> ()  [unwired: 2 in, 2 out]
        n577 = property on="Tab Control 8" class="TabCtl (strict)"("Visible"=FALSE) -> ()  [unwired: 2 in, 2 out]
        n578 = property on="Tab Control 9" class="TabCtl (strict)"("Visible"=FALSE) -> ()  [unwired: 2 in, 2 out]
        n579 = property on="Tab Control 15" class="TabCtl (strict)"("Visible"=FALSE) -> ()  [unwired: 2 in, 2 out]
        n580 = property on="Tab Control 24" class="TabCtl (strict)"("Visible"=TRUE) -> ()  [unwired: 2 in, 2 out]
        n581 = property on="Tab Control 21" class="TabCtl (strict)"("Visible"=FALSE) -> ()  [unwired: 2 in, 2 out]
        n582 = property on="Tab Control 16" class="TabCtl (strict)"("Visible"=FALSE) -> ()  [unwired: 2 in, 2 out]
        n583 = property on="Tab Control 17" class="TabCtl (strict)"("Visible"=FALSE) -> ()  [unwired: 2 in, 2 out]
        n584 = property on="Tab Control 22" class="TabCtl (strict)"("Visible"=FALSE) -> ()  [unwired: 2 in, 2 out]
        n585 = property on="Tab Control 23" class="TabCtl (strict)"("Visible"=FALSE) -> ()  [unwired: 2 in, 2 out]
        n586 = property on="Tab Control 18" class="TabCtl (strict)"("Visible"=FALSE) -> ()  [unwired: 2 in, 2 out]
        n587 = property on="Tab Control 19" class="TabCtl (strict)"("Visible"=FALSE) -> ()  [unwired: 2 in, 2 out]
        n588 = property on="Tab Control 14" class="TabCtl (strict)"("Visible"=FALSE) -> ()  [unwired: 2 in, 2 out]